vi "IMAQdx_AbsImage_Flea3_v4.7.vi"() -> ()   [LabVIEW 2013]
doc: "Take a single PixelFly exposure and display the result as an intensity graph.This VI illustrates the basics of taking an exposure with the PixelFly camera. Use Ctrl-H to get help on any of the controls\n\nCopyright 2001, The Cooke Corporation."
uses:
  LabVIEW Data V4.10/Shared Libraries/Controls/FileName_Cluster.ctl
  <vilib>/userdefined/High Color/IMAQdx.ctl
  <vilib>/vision/driver/IMAQdx.llb/IMAQdx Acquisition Mode.ctl
  Shared Libraries/Controls/FileInfo_Global.vi
  <vilib>/vision/driver/NI_Vision_Acquisition_Software.lvlib
panel:
  out "DDE Done":bool
  out "Waiting for PIXIS file":bool=TRUE
  in  "Flea Acquire":bool=TRUE
  in  "PIXIS Acquire":bool
  out "PIXIS Loop":i32=31
  out "CycleDone":bool=TRUE
  out "PIXIS Frames":i64
  in  "Interrupt":bool
  out "Status":string="Running..."
  in  "stop":bool
  in  "Tab Control":enum32{"Setup", "Images", "Hardware status"}(tab)
  in  "PIXIS Data Series Name":string="Sr_PIXIS_Seq"
  in  "Flea File Parameters":T1={"Data Root"=path "I:/Data", "Index"=3940, "Instrument"="FL3_32S2M"} {"Index" format="%04d"}
  in  "PIXIS Wave Name":string="Test_Img"
  out "PIXIS Image Note":string="Experiment=Sr\nCamera_ID=PIXIS\nImageType=Raw\nDataType=Absorption\nImageDirection=XY\nMagnification=5.480000E+0\nLastSave=dfe1ffb2f91a13864299666586c67f10630f5b22\nFileNumber=3939\nIndex=0\nIndexedWaves=BBcaptureT;BBcompT;BlueLaserBeatnote;BlueLaserLockOffset;BlueLaserProbeBN;DipAOMFreq;DipPowCr;DipPowCr2;DipPowCr3;DipPowCr4;DipPowCrFinal;DipPowHLat2;DipPowX;DipPowX2;DipPowX3;DipPowX4;DipPowXFinal;DipPowZ;DipPowZ2;DipPowZ3;DipPowZ4;DipPowZFinal;DipPowZLat;DoppCoolDet;DoppCoolStirDet;DoppCoolSweep;EOMamp;MOTPow;MOTPow2;MOTcurrent;MOTcurrent2;Nspacers;Pdet;PixisPosition;ProbeDet;ProbePow;ProbePow2;SFcoolT;SFramp;SFramp2;ShortSteckDDS;TOF;TOFaux;Vimaging;WMfreq;Xshim;XshimrMOT;Yshim;YshimrMOT;ZShimVarF;Zshim;ZshimDC;ZshimVar;ZshimrMOT;bLoadT;bMapT;bRampT;boxLoadT;boxOn;combWidthF;combWidthI;depumpOn;depumpPow;dopCoolT;dwellT;evapOn;freq;holdT;loadT;minus_zman;plus_zman;pulseLatT;rMOTbroadDetuningF;rMOTbroadDetuningI;rMOTcurrF;rMOTcurrI;rMOTon;rMOTpow2;rMOTpow3;rMOTpow4;rMOTpow5;rMOTpow6;rMOTstirDetF;rMOTstirDetI;rampLatOffT;rampLatT;rampOn;rampT;singleFreqDet;singleFreqDetF;singleFreqStirDet;singleFreqStirDetF;tEvap0;tEvap1;tEvap2;tau;tau2;varWaveP1\nIndexedValues=50.0000000000000E-3;325.000000000000E-3;374.000000000000E+3;8.75000000000000E+0;380.000000000000E+3;40.2000000000000E+6;900.000000000000E-3;1.60000000000000E+0;110.000000000000E-3;45.0000000000000E-3;200.000000000000E-3;200.000000000000E-3;1.70000000000000E+0;3.20000000000000E+0;160.000000000000E-3;80.0000000000000E-3;400.000000000000E-3;100.000000000000E-3;600.000000000000E-3;25.0000000000000E-3;15.0000000000000E-3;45.0000000000000E-3;100.000000000000E-3;-4.94000000000000E+3;-4.98000000000000E+3;-20.0000000000000E+0;8.00000000000000E+0;12.0000000000000E+0;500.000000000000E-3;-3.75000000000000E+0;-9.00000000000000E+0;4.00000000000000E+0;7.00000000000000E+0;15.3000000000000E+0;0.00000000000000E+0;3.20000000000000E+0;2.00000000000000E+0;10.0000000000000E-3;10.0000000000000E+0;15.0000000000000E+0;-50.0000000000000E+3;13.0000000000000E-3;5.00000000000000E-3;1.00000000000000E+0;0.00000000000000E+0;550.000000000000E-3;500.000000000000E-3;4.00000000000000E+0;3.20000000000000E+0;1.27500000000000E+0;1.80000000000000E+0;1.00000000000000E+0;1.27500000000000E+0;2.00000000000000E+0;3.90000000000000E+0;400.000000000000E-6;7.50000000000000E-3;1.00000000000000E+0;0.00000000000000E+0;25.0000000000000E-3;2.00000000000000E+0;0.00000000000000E+0;1.00000000000000E+0;25.0000000000000E-3;20.0000000000000E+0;1.00000000000000E+0;170.000000000000E+0;3.00000000000000E+0;40.0000000000000E-3;-7.90400000000000E+0;-9.79200000000000E+0;10.0000000000000E-6;6.47000000000000E+0;6.47000000000000E+0;-290.000000000000E-3;-200.000000000000E-3;1.00000000000000E+0;1.60000000000000E+0;7.10000000000000E+0;1.65000000000000E+0;1.25000000000000E+0;1.40000000000000E+0;6.94000000000000E+0;6.94000000000000E+0;100.000000000000E-3;100.000000000000E-3;1.00000000000000E+0;200.000000000000E-3;-6.32500000000000E+3;-5.31000000000000E+3;-6.42000000000000E+3;-5.45000000000000E+3;100.000000000000E-3;2.50000000000000E+0;4.00000000000000E+0;750.000000000000E-3;7.00000000000000E+0;2.65000000000000E+0\n# Current Variables\n#\nBBcaptureT = 5.000000E-2\nBBcompT = 3.250000E-1\nBlueDipPow = 2.400000E-1\nBlueLaserBeatnote = 3.740000E+5\nBlueLaserLockOffset = 8.750000E+0\nBlueLaserProbeBN = 3.800000E+5\nDipAOMFreq = 4.020000E+7\nDipPowCr = 9.000000E-1\nDipPowCr2 = 1.600000E+0\nDipPowCr3 = 1.100000E-1\nDipPowCr4 = 4.500000E-2\nDipPowCrFinal = 2.000000E-1\nDipPowCrTOF = 9.000000E-1\nDipPowHLat = 8.900000E-2\nDipPowHLat2 = 2.000000E-1\nDipPowX = 1.700000E+0\nDipPowX2 = 3.200000E+0\nDipPowX3 = 1.600000E-1\nDipPowX4 = 8.000000E-2\nDipPowXFinal = 4.000000E-1\nDipPowXLat = 1.000000E+0\nDipPowXTOF = 1.700000E+0\nDipPowZ = 1.000000E-1\nDipPowZ2 = 6.000000E-1\nDipPowZ3 = 2.500000E-2\nDipPowZ4 = 1.500000E-2\nDipPowZFinal = 4.500000E-2\nDipPowZLat = 1.000000E-1\nDoppCoolDet = -4.940000E+3\nDoppCoolPow = 1.250000E+0\nDoppCoolStirDet = -4.980000E+3\nDoppCoolSweep = -2.000000E+1\nDoppStirPow = 1.600000E+0\nEOMamp = 8.000000E+0\nHeatingAmp = 1.000000E-1\nHimaging = 1.000000E+0\nMOTPow = 1.200000E+1\nMOTPow2 = 5.000000E-1\nMOTcurrent = -3.750000E+0\nMOTcurrent2 = -9.000000E+0\nMOTdetuning = -4.504000E+1\nNspacers = 4.000000E+0\nPdet = 7.000000E+0\nPdet2 = 5.000000E-2\nPixisPosition = 1.530000E+1\nProbeDet = 0.000000E+0\nProbePow = 3.200000E+0\nProbePow2 = 2.000000E+0\nSFcoolT = 1.000000E-2\nSFramp = 1.000000E+1\nSFramp2 = 1.500000E+1\nShortSteckDDS = -5.000000E+4\nTOF = 1.300000E-2\nTOFaux = 5.000000E-3\nVimaging = 1.000000E+0\nWMfreq = 0.000000E+0\nXshim = 5.500000E-1\nXshimDC = 2.500000E-1\nXshimrMOT = 5.000000E-1\nYshim = 4.000000E+0\nYshimDC = 2.575000E+0\nYshimrMOT = 3.200000E+0\nZShimVarF = 1.275000E+0\nZshim = 1.800000E+0\nZshimDC = 1.000000E+0\nZshimVar = 1.275000E+0\nZshimrMOT = 2.000000E+0\nbLoadT = 3.900000E+0\nbMOToverride = 1.000000E+0\nbMapT = 4.000000E-4\nbRampT = 7.500000E-3\nboxLoadT = 1.000000E+0\nboxOn = 0.000000E+0\ncameraArmT = 5.000000E-5\ncombWidthF = 2.500000E-2\ncombWidthI = 2.000000E+0\ncompensation = -3.981000E+0\ndepumpOn = 0.000000E+0\ndepumpPow = 1.000000E+0\ndopCoolT = 2.500000E-2\ndopCoolT1 = 5.000000E-3\ndwellT = 2.000000E+1\nevapOn = 1.000000E+0\nexposureT = 1.000000E-5\nfreq = 1.700000E+2\nholdT = 3.000000E+0\nloadT = 4.000000E-2\nminus_zman = -7.904000E+0\nnumTones = 4.000000E+0\nplus_zman = -9.792000E+0\npulseLatT = 1.000000E-5\nrMOTbroadDetuningF = 6.470000E+0\nrMOTbroadDetuningI = 6.470000E+0\nrMOTcurrF = -2.900000E-1\nrMOTcurrI = -2.000000E-1\nrMOTon = 1.000000E+0\nrMOTpow1 = 7.000000E+0\nrMOTpow2 = 1.600000E+0\nrMOTpow3 = 7.100000E+0\nrMOTpow4 = 1.650000E+0\nrMOTpow5 = 1.250000E+0\nrMOTpow6 = 1.400000E+0\nrMOTstirDetF = 6.940000E+0\nrMOTstirDetI = 6.940000E+0\nrampLatOffT = 1.000000E-1\nrampLatT = 1.000000E-1\nrampOn = 1.000000E+0\nrampT = 2.000000E-1\nsingleFreqDet = -6.325000E+3\nsingleFreqDetF = -5.310000E+3\nsingleFreqStirDet = -6.420000E+3\nsingleFreqStirDetF = -5.450000E+3\nstirWidthF = 2.500000E-2\nstirWidthI = 2.000000E+0\ntEvap0 = 1.000000E-1\ntEvap1 = 2.500000E+0\ntEvap2 = 4.000000E+0\ntau = 7.500000E-1\ntau2 = 7.000000E+0\nvarWaveP1 = 2.650000E+0\nvarWaveP2 = 1.200000E+0\n#\n# Master Staging List\n#Comment\tMarker\tMode\tGroup\tDelay\tX ODT Shuttter\tX ODT AO TTL\tVert ODT Shutter\tVert ODT AO TTL\tCross ODT Shutter\tCross ODT AO TTL\t707s Shutter\t\tH Probe AO TTL\tFreq Switch rMOT\trMOT AO TTL\t\tTrans AO TTL\tV Probe AO TTL\tZman AO TTL\tbMOT AO TTL\t60 Hz Trig Gate\tWindow Heater TTL\tPB_18\t\tPB_20 Trigger Dev3\tPB_21 Trigger Dev2\tPB_22 Trigger Dev1\tPB_23 Trigger Dev0\tStep\t~Atomic Beam Shutter\tGate Valve\tDO0_2\tShortSteck Shutter\t~Zman Coils\t~ MOT Coils\t~ Dipole Flea3 Shutter\trMOT Shutter\t+Zeeman Coils\t-Zeeman Coils\tCompensation Coils\tMOT Coils\trMOT AO Power\trMOT Freq Amplitude\trMOT Freq Offset\tH Lattice AO Power\tTrans Shutter\tV Probe Shutter\tZman Shutter\tbMOT Shutter\tGrassHp Trig\t679 Shutter\t~Pixis Shutter\t~Abs Flea3 Shutter\tDMD TTL Trigger\tMOT AO Power\tProbe AO Power\tAO1_3\tX Shim Coils\tY Shim Coils\tZ Shim Coils\tVert ODT AO Power\tPIXIS Ext Shutter\tZeeman Laser Shutter\tBlueODT Shutter\tH Probe Shutter\tH Lattice Shutter\tH Lattice AO TTL\tParametric Heating\t689c AOM TTL\tAO2_0\tAO2_1\tD03_0\tD03_1\tD03_2\tD03_3\tD03_4\tD03_5\tD03_6\tD03_7\trMOT Stir Freq Offset\tBlueODT Power\tCrossODT Power\tVariable Waveplate\tH Probe AO Pow\tAO3_5\trMOT Stir Power\tX ODT AO Power\tSRS Freq\tSRS Amp\tSRS Offset\tSRS Func Type\tRedMotDDS\tRedMotDDS_ 0\tRedMotDDS_ 1\tRedMotDDS_ 2\tStirringDDS\tStirringDDS_ 0\tStirringDDS_ 1\tStirringDDS_ 2\tBlueBN\tBlueBN_ 0\tSSteckBN\tSSteckBN_ 0\tPosition\tRun Mode\tDDS\tDDS_ 0\tDDS_ 1\tDDS_ 2\tDDS_ 3\tDDS_ 4\tDDS_ 5\tDDS_ 6\tDDS_ 7\tDDS_ 8\tDDS_ 9\tDDS_ 10\tDDS_ 11\tDDS_ 12\tDDS_ 13\tDDS_ 14\tDDS_ 15\tDDS_ 16\tDDS_ 17\tFunction\tArg_0\tArg_1\tArg_2\tArg_3\r\n\r\nreset\t\tRamp\t1\t.1\t1\t1\t1\t1\t1\t1\t1\t0\t1\t0\t1\t0\t1\t1\t1\t1\t0\t0\t0\t0\t0\t0\t0\t0\t0\t0\t1\t0\t0\t0\t0\t1\t0\tplus_zman\tminus_zman\tcompensation\tMOTcurrent\trMOTpow1\tcombAmplitude(combWidthI)\trMOTdelta(-(rMOTbroadDetuningI +combWidthI/2))\tODTpowHLat(DipPowHLat2)\t0\t0\t1\t0\t1\t1\t1\t1\t5\tbMOTpow(0.5)\tProbePow\t0\tXshim\tYshim\tZshim\tODTpowZ(DipPowZ)\t0\t0\t0\t0\t0\t1\t0\t1\t0\t0\t0\t0\t0\t0\t0\t0\t0\t0\trMOTdelta(-(rMOTstirDetI +stirWidthI/2))\tODTpowBlue(.05)\tODTpowXY(DipPowCr)\tvarWaveP1\tProbePow2\tAmp688(depumpPow)\trMOTpow3\tODTpowX(DipPowX)\tfreq\tHeatingAmp\t0\tSine\tDetuning\tsingleFreqDet\t-20\t8\tDetuning\tsingleFreqStirDet\t0\t0\tBlueBN\tBlueLaserBeatnote\tSSteckBN\tShortSteckDDS\tPixisPos(TOF)\tCycle Wait for Move\tMultipleFreqs2\t655\t12\t1240\t9\t1510\t11\t1720\t8\tfreq\tEOMamp\t10\t0\t10\t0\t10\t0\tnumTones\tdwellT\tboxPattern\t25\t11.5\t200\t96\r\nblue MOT load\t\tRamp\t1\tbLoadT\t1\t1\t1\t1\t1\t1\t1\t0\t1\t0\t1\t0\t1\t1\t1\t1\t0\t1\t0\t0\t0\t0\t0\t0\t0\t0\t1\t1\t0\t0\t0\t1\t1\tplus_zman\tminus_zman\tcompensation\tMOTcurrent\trMOTpow1\tcombAmplitude(combWidthI)\trMOTdelta(-(rMOTbroadDetuningI +combWidthI/2))\tODTpowHLat(DipPowHLat)\t1\t0\t1\tbMOToverride\t1\t1\t1\t1\t0\tbMOTpow(MOTPow)\tProbePow\t0\tXshim\tYshim\tZshim\tODTpowZ(DipPowZ)\t0\t1\t1\t0\t0\t1\t0\t0\t0\t0\t0\t0\t0\t0\t0\t0\t0\t0\trMOTdelta(-(rMOTstirDetI +stirWidthI/2))\tODTpowBlue(0.05)\tODTpowXY(DipPowCr)\tvarWaveP1\tProbePow2\tAmp688(depumpPow)\trMOTpow3\tODTpowX(DipPowX)\tfreq\tHeatingAmp\t0\tSine\tDetuning\tsingleFreqDet\t-20\t8\tDetuning\tsingleFreqStirDet\t0\t0\tBlueBN\tBlueLaserBeatnote\tSSteckBN\tShortSteckDDS\tPixisPos(TOF)\tCycle Wait for Move\t0\t0\t0\t0\t0\t0\t0\t0\t0\t0\t0\t0\t0\t0\t0\t0\t0\t0\t0\t0\t0\t0\t0\t0\r\npretrig\t\tRamp\t1\t6.244m\t1\t1\t1\t1\t1\t0\t1\t0\t1\t0\t1\t0\t1\t1\t1\t1\t0\t1\t0\t0\t0\t0\t0\t0\t0\t0\t1\t1\t0\t0\t0\t0\t1\tplus_zman\tminus_zman\tcompensation\tMOTcurrent\trMOTpow1\tcombAmplitude(combWidthI)\trMOTdelta(-(rMOTbroadDetuningI +combWidthI/2))\tODTpowHLat(.6)\t1\t0\t1\tbMOToverride\t0\t1\t0\t0\t0\tbMOTpow(MOTPow)\tProbePow\t0\tXshim\tYshim\tZshim\tODTpowZ(DipPowZ)\t0\t1\t1\t0\t0\t1\t0\t1\t0\t0\t0\t0\t0\t0\t0\t0\t0\t0\trMOTdelta(-(rMOTstirDetI +stirWidthI/2))\tODTpowBlue(.05)\tODTpowXY(DipPowCr)\tvarWaveP1\tProbePow2\tAmp688(depumpPow)\trMOTpow3\tODTpowX(DipPowX)\tfreq\tHeatingAmp\t0\tSine\tDetuning\tsingleFreqDet\t-20\t8\tDetuning\tsingleFreqStirDet\t0\t0\tBlueBN\tBlueLaserBeatnote\tSSteckBN\tShortSteckDDS\tPixisPos(TOF)\tCycle Wait for Move\t0\t0\t0\t0\t0\t0\t0\t0\t0\t0\t0\t0\t0\t0\t0\t0\t0\t0\t0\t0\t0\t0\t0\t0\r\nblue MOT load\t\tRamp\t0\tbLoadT\t1\t1\t1\t1\t1\t1\t1\t0\t1\t0\t1\t0\t1\t1\t1\t1\t0\t0\t0\t0\t0\t0\t0\t0\t0\t0\t1\t1\t0\t0\t0\t1\t1\tplus_zman\tminus_zman\tcompensation\tMOTcurrent\trMOTpow1\tcombAmplitude(combWidthI)\trMOTdelta(-(rMOTbroadDetuningI +combWidthI/2))\tODTpowHLat(DipPowHLat)\t1\t0\t1\tbMOToverride\t1\t1\t1\t1\t0\tbMOTpow(MOTPow)\tProbePow\t0\tXshim\tYshim\tZshim\tODTpowZ(DipPowZ)\t0\t1\t0\t0\t0\t1\t0\t1\t0\t0\t0\t0\t0\t0\t0\t0\t0\t0\trMOTdelta(-(rMOTstirDetI +stirWidthI/2))\tODTpowBlue(0)\tODTpowXY(DipPowCr)\tvarWaveP1\tProbePow2\tAmp688(depumpPow)\trMOTpow3\tODTpowX(DipPowX)\tfreq\tHeatingAmp\t0\tSine\tDetuning\tsingleFreqDet\t-20\t8\tDetuning\tsingleFreqStirDet\t0\t0\tBlueBN\tBlueLaserBeatnote\tSSteckBN\tShortSteckDDS\tPixisPos(TOF)\tCycle Wait for Move\t0\t0\t0\t0\t0\t0\t0\t0\t0\t0\t0\t0\t0\t0\t0\t0\t0\t0\t0\t0\t0\t0\t0\t0\r\ndump bMOT\t\tRamp\t1\t0.1-bRampT\t1\t1\t1\t1\t1\t1\t1\t0\t1\t0\t1\t0\t1\t1\t1\t1\t0\t1\t0\t0\t0\t0\t0\t0\t1m\t0\t1\t1\t0\t0\t0\t1\t1\tplus_zman\tminus_zman\tcompensation\tMOTcurrent\trMOTpow1\tcombAmplitude(combWidthI)\trMOTdelta(-(rMOTbroadDetuningI +combWidthI/2))\tODTpowHLat(DipPowHLat)\t1\t0\t1\tbMOToverride\t1\t1\t1\t1\t0\tbMOTpow(MOTPow)\tProbePow\t0\tXshim\tYshim\tZshim\tODTpowZ(DipPowZ)\t0\t1\t0\t0\t0\t1\t0\t1\t0\t0\t0\t0\t0\t0\t0\t0\t0\t0\trMOTdelta(-(rMOTstirDetI +stirWidthI/2))\tODTpowBlue(0)\tODTpowXY(DipPowCr)\tvarWaveP1\tProbePow2\tAmp688(depumpPow)\trMOTpow3\tODTpowX(DipPowX)\tfreq\tHeatingAmp\t0\tSine\tDetuning\tsingleFreqDet\t-20\t8\tDetuning\tsingleFreqStirDet\t0\t0\tBlueBN\tBlueLaserBeatnote\tSSteckBN\tShortSteckDDS\tPixisPos(TOF)\tCycle Wait for Move\t0\t0\t0\t0\t0\t0\t0\t0\t0\t0\t0\t0\t0\t0\t0\t0\t0\t0\t0\t0\t0\t0\t0\t0\r\ndump bMOT\t\tRamp\t1\tbRampT\t1\t1\t1\t1\t1\t1\t1\t0\t1\t0\t1\t0\t1\t1\t1\t1\t0\t1\t0\t0\t0\t0\t0\t0\t1m\t0\t1\t0\t0\t0\t0\t1\t1\tplus_zman\tminus_zman\tcompensation\tLineRamp(f,MOTcurrent,MOTcurrent2)\trMOTpow1\tcombAmplitude(combWidthI)\trMOTdelta(-(rMOTbroadDetuningI +combWidthI/2))\tODTpowHLat(DipPowHLat)\t1\t0\t1\tbMOToverride\t1\t1\t1\t1\t0\tLineRamp(f,bMOTpow(MOTPow),bMOTpow(MOTPow2))\tProbePow\t0\tLineRamp(f,Xshim,XshimrMOT)\tLineRamp(f,Yshim,YshimrMOT)\tLineRamp(f,Zshim,ZshimrMOT)\tODTpowZ(DipPowZ)\t0\t0\t0\t0\t0\t1\t0\t1\t0\t0\t0\t0\t0\t0\t0\t0\t0\t0\trMOTdelta(-(rMOTstirDetI +stirWidthI/2))\tODTpowBlue(0)\tODTpowXY(DipPowCr)\tvarWaveP1\tProbePow2\tAmp688(depumpPow)\trMOTpow3\tODTpowX(DipPowX)\tfreq\tHeatingAmp\t0\tSine\tDetuning\tsingleFreqDet\t-20\t8\tDetuning\tsingleFreqStirDet\t0\t0\tBlueBN\tBlueLaserBeatnote\tSSteckBN\tShortSteckDDS\tPixisPos(TOF)\tCycle Wait for Move\t0\t0\t0\t0\t0\t0\t0\t0\t0\t0\t0\t0\t0\t0\t0\t0\t0\t0\t0\t0\t0\t0\t0\t0\r\nCamWaitTime\t\tRamp\t0\t.1\t1\t1\t1\t1\t1\t1\t1\t0\t0\t0\t1\t0\t1\t0\t1\t1\t0\t1\t0\t0\t0\t0\t0\t0\t0\t0\t1\t0\t0\t0\t0\t1\t1\tplus_zman\tminus_zman\tcompensation\tMOTcurrent\trMOTpow1\tcombAmplitude(combWidthI)\trMOTdelta(-(rMOTbroadDetuningI +combWidthI/2))\tODTpowHLat(DipPowHLat)\t1\t0\t1\tbMOToverride\t1\t1\t1\t1\t0\tbMOTpow(MOTPow2)\tProbePow\t0\tXshimrMOT\tYshimrMOT\tZshimrMOT\tODTpowZ(DipPowZ)\t0\t0\t0\t0\t0\t1\t0\t0\t0\t0\t0\t0\t0\t0\t0\t0\t0\t0\trMOTdelta(-(rMOTstirDetI +stirWidthI/2))\tODTpowBlue(0)\tODTpowXY(DipPowCr)\tvarWaveP1\tProbePow2\tAmp688(depumpPow)\trMOTpow3\tODTpowX(DipPowX)\tfreq\tHeatingAmp\t0\tSine\tDetuning\tsingleFreqDet\t-20\t8\tDetuning\tsingleFreqStirDet\t0\t0\tBlueBN\tBlueLaserBeatnote\tSSteckBN\tShortSteckDDS\tPixisPos(TOF)\tCycle Wait for Move\t0\t0\t0\t0\t0\t0\t0\t0\t0\t0\t0\t0\t0\t0\t0\t0\t0\t0\t0\t0\t0\t0\t0\t0\r\nProbeShutOn\t\tRamp\t1-rMOTon\t1120e-6\t1\t1\t1\t1\t1\t1\t1\t0\t0\t0\t1\t0\t0\t0\t0\t1\t0\t1\t0\t0\t0\t0\t0\t0\t0\t1\t1\t0\t0\t0\t0\t1\t1\tplus_zman\tminus_zman\tcompensation\tMOTcurrent\trMOTpow1\tcombAmplitude(combWidthI)\trMOTdelta(-(rMOTbroadDetuningI +combWidthI/2))\tODTpowHLat(DipPowHLat)\t1\t0\t1\tbMOToverride\t1\t1\t1\t1\t0\tbMOTpow(MOTPow2)\tProbePow\t0\tXshimrMOT\tYshimrMOT\tZshimrMOT\tODTpowZ(DipPowZ)\t0\t0\t0\tHimaging\t0\t1\t0\t1\t0\t0\t0\t0\t0\t0\t0\t0\t0\t0\trMOTdelta(-(rMOTstirDetI +stirWidthI/2))\tODTpowBlue(0)\tODTpowXY(DipPowCr)\tvarWaveP1\tProbePow2\tAmp688(depumpPow)\trMOTpow3\tODTpowX(DipPowX)\tfreq\tHeatingAmp\t0\tSine\tDetuning\tsingleFreqDet\t-20\t8\tDetuning\tsingleFreqStirDet\t0\t0\tBlueBN\tBlueLaserBeatnote\tSSteckBN\tShortSteckDDS\tPixisPos(TOF)\tCycle Wait for Move\t0\t0\t0\t0\t0\t0\t0\t0\t0\t0\t0\t0\t0\t0\t0\t0\t0\t0\t0\t0\t0\t0\t0\t0\r\nRepumpShutOff\t\tRamp\t1-rMOTon\t260e-6\t1\t1\t1\t1\t1\t1\t1\t0\t0\t0\t1\t0\t0\t0\t0\t1\t0\t1\t0\t0\t0\t0\t0\t0\t0\t1\t1\t0\t0\t0\t0\t1\t1\tplus_zman\tminus_zman\tcompensation\tMOTcurrent\trMOTpow1\tcombAmplitude(combWidthI)\trMOTdelta(-(rMOTbroadDetuningI +combWidthI/2))\tODTpowHLat(DipPowHLat)\t1\t0\t0\tbMOToverride\t1\t1\t1\t1\t0\tbMOTpow(MOTPow2)\tProbePow\t0\tXshimrMOT\tYshimrMOT\tZshimrMOT\tODTpowZ(DipPowZ)\t0\t0\t0\tHimaging\t0\t1\t0\t1\t0\t0\t0\t0\t0\t0\t0\t0\t0\t0\trMOTdelta(-(rMOTstirDetI +stirWidthI/2))\tODTpowBlue(0)\tODTpowXY(DipPowCr)\tvarWaveP1\tProbePow2\tAmp688(depumpPow)\trMOTpow3\tODTpowX(DipPowX)\tfreq\tHeatingAmp\t0\tSine\tDetuning\tsingleFreqDet\t-20\t8\tDetuning\tsingleFreqStirDet\t0\t0\tBlueBN\tBlueLaserBeatnote\tSSteckBN\tShortSteckDDS\tPixisPos(TOF)\tCycle Wait for Move\t0\t0\t0\t0\t0\t0\t0\t0\t0\t0\t0\t0\t0\t0\t0\t0\t0\t0\t0\t0\t0\t0\t0\t0\r\nMOTShutOff\t\tRamp\t1-rMOTon\t1370e-6\t1\t1\t1\t1\t1\t1\t1\t0\t0\t0\t1\t0\t0\t0\t0\t1\t0\t1\t0\t0\t0\t0\t0\t0\t0\t1\t1\t0\t0\t0\t0\t1\t1\tplus_zman\tminus_zman\tcompensation\tMOTcurrent\trMOTpow1\tcombAmplitude(combWidthI)\trMOTdelta(-(rMOTbroadDetuningI +combWidthI/2))\tODTpowHLat(DipPowHLat)\t1\t0\t0\t0\t1\t1\t1\t1\t0\tbMOTpow(MOTPow2)\tProbePow\t0\tXshimrMOT\tYshimrMOT\tZshimrMOT\tODTpowZ(DipPowZ)\t0\t0\t0\tHimaging\t0\t1\t0\t1\t0\t0\t0\t0\t0\t0\t0\t0\t0\t0\trMOTdelta(-(rMOTstirDetI +stirWidthI/2))\tODTpowBlue(0)\tODTpowXY(DipPowCr)\tvarWaveP1\tProbePow2\tAmp688(depumpPow)\trMOTpow3\tODTpowX(DipPowX)\tfreq\tHeatingAmp\t0\tSine\tDetuning\tsingleFreqDet\t-20\t8\tDetuning\tsingleFreqStirDet\t0\t0\tBlueBN\tBlueLaserBeatnote\tSSteckBN\tShortSteckDDS\tPixisPos(TOF)\tCycle Wait for Move\t0\t0\t0\t0\t0\t0\t0\t0\t0\t0\t0\t0\t0\t0\t0\t0\t0\t0\t0\t0\t0\t0\t0\t0\r\nCoil Switch\t\tRamp\trMOTon\t220e-6\t1\t1\t1\t1\t1\t1\t1\t0\t1\t0\t1\t0\t0\t1\t0\t1\t0\t1\t0\t0\t0\t0\t0\t0\t0\t1\t1\t0\t0\t0\t0\t1\t1\tplus_zman\tminus_zman\tcompensation\trMOTcurrI\trMOTpow1\tcombAmplitude(combWidthI)\trMOTdelta(-(rMOTbroadDetuningI +combWidthI/2))\tODTpowHLat(DipPowHLat)\t1\t0\t0\t0\t1\t1\t1\t1\t0\tbMOTpow(2)\tProbePow\t0\tXshimrMOT\tYshimrMOT\tZshimrMOT\tODTpowZ(DipPowZ)\t0\t0\t0\t0\t0\t1\t0\t1\t0\t0\t0\t0\t0\t0\t0\t0\t0\t0\trMOTdelta(-(rMOTstirDetI +stirWidthI/2))\tODTpowBlue(0)\tODTpowXY(DipPowCr)\tvarWaveP1\tProbePow2\tAmp688(depumpPow)\trMOTpow3\tODTpowX(DipPowX)\tfreq\tHeatingAmp\t0\tSine\tDetuning\tsingleFreqDet\t-20\t8\tDetuning\tsingleFreqStirDet\t0\t0\tBlueBN\tBlueLaserBeatnote\tSSteckBN\tShortSteckDDS\tPixisPos(TOF)\tCycle Wait for Move\t0\t0\t0\t0\t0\t0\t0\t0\t0\t0\t0\t0\t0\t0\t0\t0\t0\t0\t0\t0\t0\t0\t0\t0\r\n60HzTrigger\t\tHalt\t0\t10u\t1\t1\t1\t1\t1\t1\t1\t0\t0\t0\t1\t0\t0\t0\t0\t0\t0\t1\t0\t0\t0\t0\t0\t0\t0\t1\t1\t0\t0\t0\t0\t1\t1\tplus_zman\tminus_zman\tcompensation\trMOTcurrI\trMOTpow1\tcombAmplitude(combWidthI)\trMOTdelta(-(rMOTbroadDetuningI +combWidthI/2))\tODTpowHLat(DipPowHLat)\t1\t0\t0\t0\t1\t1\t1\t1\t0\tbMOTpow(2)\tProbePow\t0\tXshimrMOT\tYshimrMOT\tZshimrMOT\tODTpowZ(DipPowZ)\t0\t0\t0\t0\t0\t1\t0\t1\t0\t0\t0\t0\t0\t0\t0\t0\t0\t0\trMOTdelta(-(rMOTstirDetI +stirWidthI/2))\tODTpowBlue(0)\tODTpowXY(DipPowCr)\tvarWaveP1\tProbePow2\tAmp688(depumpPow)\trMOTpow3\tODTpowX(DipPowX)\tfreq\tHeatingAmp\t0\tSine\tDetuning\tsingleFreqDet\t-20\t8\tDetuning\tsingleFreqStirDet\t0\t0\tBlueBN\tBlueLaserBeatnote\tSSteckBN\tShortSteckDDS\tPixisPos(TOF)\tCycle Wait for Move\t0\t0\t0\t0\t0\t0\t0\t0\t0\t0\t0\t0\t0\t0\t0\t0\t0\t0\t0\t0\t0\t0\t0\t0\r\nCapture Red MOT\t\tRamp\trMOTon\tBBcaptureT\t1\t1\t1\t1\t1\t1\t1\t0\t1\t0\t1\t0\t0\t1\t0\t0\t0\t1\t0\t0\t0\t0\t0\t0\t1m\t1\t1\t0\t0\t0\t0\t1\t1\tplus_zman\tminus_zman\tcompensation\trMOTcurrI\trMOTpow1\tcombAmplitude(combWidthI)\trMOTdelta(-(rMOTbroadDetuningI +combWidthI/2))\tODTpowHLat(DipPowHLat)\t0\t0\t0\t0\t1\t1\t1\t1\t0\tbMOTpow(0.5)\tProbePow\t0\tXshimrMOT\tYshimrMOT\tZshimrMOT\tODTpowZ(DipPowZ)\t0\t0\t0\t0\t0\t1\t0\t1\t0\t0\t0\t0\t0\t0\t0\t0\t0\t0\trMOTdelta(-(rMOTstirDetI +stirWidthI/2))\tODTpowBlue(0)\tODTpowXY(DipPowCr)\tvarWaveP1\tProbePow2\tAmp688(depumpPow)\trMOTpow3\tODTpowX(DipPowX)\tfreq\tHeatingAmp\t0\tSine\tDetuning\tsingleFreqDet\t-20\t8\tDetuning\tsingleFreqStirDet\t0\t0\tBlueBN\tBlueLaserProbeBN\tSSteckBN\tShortSteckDDS\tPixisPos(TOF)\tCycle Wait for Move\t0\t0\t0\t0\t0\t0\t0\t0\t0\t0\t0\t0\t0\t0\t0\t0\t0\t0\t0\t0\t0\t0\t0\t0\r\nRamp Red MOT\t\tRamp\trMOTon\tBBcompT\t1\t1\t1\t1\t1\t1\t1\t0\t1\t0\t1\t0\t0\t1\t0\t0\t0\t1\t0\t0\t0\t0\t0\t0\t10u\t1\t1\t0\t0\t0\t0\t1\t1\tplus_zman\tminus_zman\tcompensation\tLineRamp(f,rMOTcurrI,rMOTcurrF)\tHalfGaussRamp(t,rMOTpow1,rMOTpow2, BBcompT)\tLineRamp(f,combAmplitude(combWidthI),combAmplitude(combWidthF))\tLineRamp(f,rMOTdelta(-(rMOTbroadDetuningI +combWidthI/2)),rMOTdelta(-(rMOTbroadDetuningF +combWidthF/2)))\tODTpowHLat(DipPowHLat)\t0\t0\t0\t0\t1\t1\t1\t1\t0\tbMOTpow(0.5)\tProbePow\t0\tXshimrMOT\tYshimrMOT\tLineRamp(f,ZshimrMOT,ZshimVar)\tODTpowZ(DipPowZ)\t0\t0\t0\t0\t0\t1\t0\t1\t0\t0\t0\t0\t0\t0\t0\t0\t0\t0\tLineRamp(f,rMOTdelta(-(rMOTstirDetI +stirWidthI/2)),rMOTdelta(-(rMOTstirDetF +stirWidthF/2)))\tODTpowBlue(0)\t